vi "for testing.vi"() -> ()   [LabVIEW 2016]
uses:
  C:/Users/Anatec i3/Desktop/Labview Projects/IR OPO Controller/Branches/XPS version/uc480DotNet.dll
  uc480DotNet.dll
  <vilib>/Utility/miscctls.llb/LVBoundsTypeDef.ctl
  <vilib>/Utility/config.llb/Write Key (Double).vi
  <vilib>/Utility/config.llb/Write Key (I32).vi
  <vilib>/Utility/config.llb/Read Key (String).vi
  <vilib>/Utility/config.llb/Read Key (Double).vi
  <vilib>/Utility/config.llb/Read Key (I32).vi
  <vilib>/Utility/config.llb/NI_LVConfig.lvlib
  <vilib>/vision/NI_Vision_Development_Module.lvlib
  System.Windows.Forms
panel:
  out "[0]":i32
  out "x*y":dbl
  out "Image Pixels (U8)":u8[][](array[numeric])
  out "ROI width":dbl
  out "Lines":dbl
  out "height step size":dbl
  out "Xspot diam":dbl
  out "Y spot diam":dbl
  out "Process time":dbl=117.0
  in  "Width (µm)":i32=240
  in  "Y offset":i32=406 step=1
  in  "X offset":i32=693 step=1
  in  "Processing time unit":string(combo)="sec"
  in  "EXIT 2":bool
  in  "Camera":refnum<k24>(container)
  in  "Init Camera":bool
  in  "Start Live":bool
  in  "Stop Live":bool
  in  "Load Parameter":bool
  out "Error Out":errorcluster caption="error"
  out "Bits/Pixel":i32=32
  out "Width":i32=1280
  out "Height":i32=1024
  out "Serial Number":string="4102944807"
  in  "Camera ID":i32
  in  "Mode":i32(ring) items=["RGB 32"=0, "RGB 24"=1, "Y8 Monochrom"=6]
  in  "Zoom":dbl(ring)=1.5 items=["4X"=4.0, "2X"=2.0, "1.5X"=1.5, "1.25X"=1.25, "1X"=1.0]
  in  "Gain Boost":bool=TRUE
  in  "Snapshot":bool
  out "Output":picture
  out "Source":T1(plugin-control)
  in  "Exposure":dbl(slide)=99.80425000000001 min=0.06241666666666667 max=99.80425000000001 step=0.06241666666666667 scale=0.06241666666666667..99.80425000000001 scale format="%#.3g"
  in  "Framerate":dbl(slide)=10.002522802986672 min=0.47411700449083627 max=15.001275108384213 step=0.014032998230481021 scale=0.47411700449083627..15.001275108384213 scale format="%#.3g"
  in  "Pixelclock":i32(slide)=24 min=5 max=40 step=1 scale=5.0..40.0
  in  "Exit Camera":bool
  out "Camera Status":string="Load parameter"
  out "Log":string
  out "Y Step size in µm":i32=121
  out "Time array":dbl[][](array[numeric])
  out "ROI container\nheigth (µm)":i32=2267
  out "ROI container\nwidth (µm)":i32=2267
  out "Processi time (sec)":i32=117
  out "ROI Rectangle X position":i32=594
  out "Commands array":string[][](array[string])
  out "Laser on/off array":bool[][](array[boolean])
  out "ROI Area \n(mm2)":dbl=4.035870075999999
  out "Axis 1 Offset":dbl
  out "Axis 2 Offset":dbl
  out "ROI Rectangle Y Position":i32
  in  "Precision (%)":dbl=0.9 min=0.0 max=1.0 step=0.01 format="%#_13g"
  in  "Process Image":bool
  in  "EXIT 3":bool
  in  "Pixel size":dbl=12.19 step=0.01
  in  "Speed (µm/s)":i32=1000
  in  "Heigth (µm)":i32=240
  in  "Height  step \ndivider":i32=2
  in  "Wavelength":dbl=2940.0 min=2600.0 max=3200.0 step=1.0
  in  "Axis Initial Parameters":T2={"Velocity (units/seconds)"=1.0, "Acceleration (units/seconds²)"=20.0, "Minimum Jerk Time (seconds)"=0.005, "Maximum Jerk Time (seconds)"=0.009} {"Maximum Jerk Time (seconds)" format="%.6e"; "Minimum Jerk Time (seconds)" format="%.6e"; "Acceleration (units/seconds²)" format="%.6e"; "Velocity (units/seconds)" format="%.6e"}
  out "Axis 1":string
  out "Axis 2":string
  out "Default Wavelenght":i32
  out "XPS_Address":string
  out "Velocity":dbl
  out "Acceleration":dbl
  in  "Repetition \nRate":enum16{"1", "2", "5", "10", "20"}(ring)=enum."20"
  in  "Flash lamp - Q Switch delay (%)":i16(slide) min=0 max=100 scale=0.0..100.0 scale format="%#.1f"
  in  "Capture":bool
  in  "Log Capture":bool
  in  "Acceleration \n(mm/s²)":dbl=20.0
  in  "Transparency":u8 max=80 step=1
  in  "Home Axes":bool
  in  "Axes Manual Control":bool
  in  "Save configuration":bool
  in  "Stages status":bool
  in  "Open \nManual":bool
  in  "Alignment \ndiode":bool
  in  "Overlay MSI Image":bool
  in  "EXIT":bool
  in  "Tune":bool
  out "Laser Operation":bool
  in  "LASER":bool
  in  "LAMP":bool
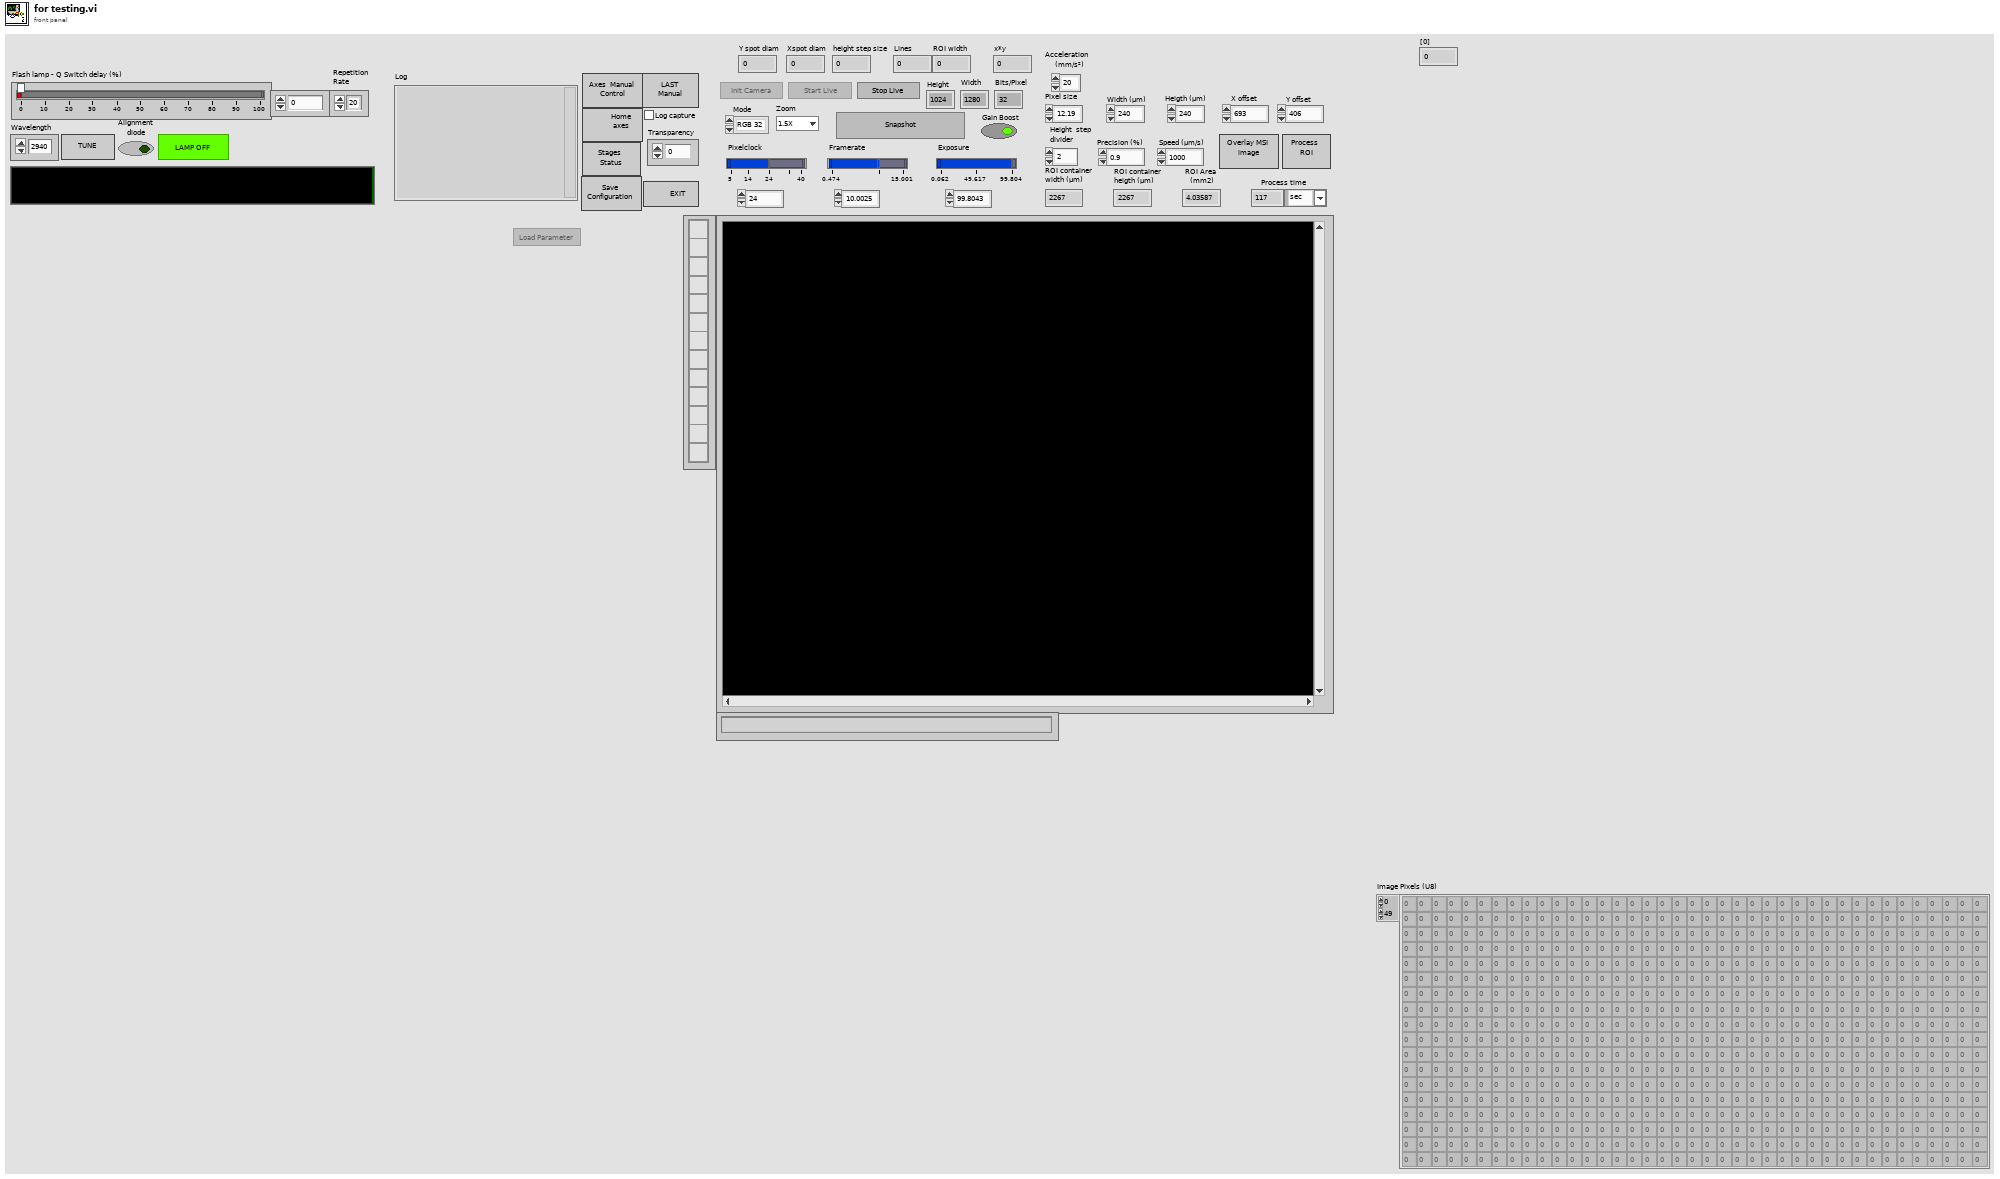
[diagram p1: front panel]
types:
  T1 = typedef "IMAQ Image.ctl" = refnum<image>
  T2 = cluster{"Velocity (units/seconds)":dbl, "Acceleration (units/seconds²)":dbl, "Minimum Jerk Time (seconds)":dbl, "Maximum Jerk Time (seconds)":dbl}
  T3 = typedef "Image Type" = u32
  T4 = cluster{"Global Rectangle":i32[], "Contours":cluster{"Contour Type":u32, "ROI Type":u32, "Points":i32[]}[]}
  T5 = typedef "NI_LVConfig.lvlib/Config Data RefNum.ctl" = refnum<k1>
  T6 = cluster{"connection TCP":refnum<k5>, "LogTo File":bool, "Log File refnum":refnum<file>, "no error if error log":bool}
  T7 = typedef "LVBoundsTypeDef.ctl" = cluster{"Width":u32, "Height":u32}
  T8 = enum8{"Enabled", "Disabled", "Disabled and Grayed Out"}
  T9 = enum16{"Initialize", "Lamp ON", "Lamp OFF", "Q-switch ON", "Q-switch OFF", "Adjust Energy", "Change Rep. Rate", "Send String"}
  T10 = enum16{"open", "replace", "create", "open or create", "replace or create", "replace or create with confirmation"}
  T11 = enum32{"Invalid", "Standard", "Closed", "Hidden", "Minimized", "Maximized"}
  T12 = enum32{"invalid app kind", "Development System", "Run Time System", "Student Edition", "Embedded LabVIEW", "Evaluation", "Custom"}
diagram:
  w16 = 1 items=["None", "FixedSingle", "Fixed3D"] ("BorderStyle")
  # "Camera control buttons"
  # "Button and controls"
  n1 = while "ROI Processing" {
    stop <- w52 stop-if-true
    n2 = event shown="[1] \"Process Image\": Value Change" {
      selector: _ -> [_ _]
      dyn-events: _ -> [_ _]
      timeout: _ -> [_ _]
      tunnel: ["EXIT 3" _] -> w52
      tunnel: [_ w58] -> w45
      event "EXIT": Value Change {
        n3 = event-data() -> ()  [unwired: 1 in, 6 out]
      }
      event "Process Image": Value Change {
        n4 = event-data() -> ()  [unwired: 1 in, 6 out]
        n5 = case shown="True" "Process Image" {
          tunnel: ["" "Processing done"] -> w58
          frame False {
          }
          frame True {
            w72 = 0.2  # Delay after laser on/off
            w84 = 2.0 ("y")
            w131 = T3 0 items=["Grayscale (U8)", "Grayscale (I16)", "Grayscale (SGL)", "Complex (CSG)", "RGB (U32)", "HSL (U32)", "RGB (U64)", "Grayscale (U16)"] ("Image Type")
            w134 = i16 3 ("precision (6)")
            w124 = 1000 ("y")
            n6 = local read "Source"() -> (w133:T1)
            n7 = property on="Source" class="ImageControl"() -> ("ROI"=w140:T4)  [unwired: 2 in, 2 out]
            n8 = call "IMAQ Cast Image"("Image Type"=w131, "Image Src"=w133) -> ("Image Dst Out"=w132:T1)  [unwired: 8 in, 1 out]
            n9 = Unbundle By Name(w140) -> ("Global Rectangle"=w139:i32[])
            n10 = call "IMAQ ROIToMask 2"("ROI Descriptor"=w140, "Image"=w132) -> ("Image Out"=w142:T1)  [unwired: 7 in, 2 out]
            n11 = local read "Heigth (µm)"() -> (w93:i32)
            n12 = local read "Width (µm)"() -> (w92:i32)
            n13 = local read "X offset"() -> (w127:i32)
            n14 = local read "Y offset"() -> (w129:i32)
            n15 = call "IMAQ ImageToArray"("Image"=w142) -> ("Image Pixels (U8)"=w114:u8[][])  [unwired: 3 in, 4 out]
            "Image Pixels (U8)" <- w114
            n16 = Index Array(array=w139, index=0) -> (element=w128:i32)
            "ROI Rectangle X position" <- w128
            n17 = Index Array(array=w139, index=1) -> (element=w130:i32)
            "ROI Rectangle Y Position" <- w130
            n18 = Divide "X spot radius in micron"(x=w92, y=w84) -> (x/y=w96:dbl)
            n19 = Divide "Y spot radius in micron"(x=w93, y=w84) -> (x/y=w95:dbl)
            n20 = Empty Array?(array=w114) -> (empty?=w115:bool)
            n21 = Subtract(x=w128, y=w127) -> (x-y=w136:i32)
            n22 = Subtract(x=w130, y=w129) -> (x-y=w135:i32)
            n23 = case shown="False" w115 {
              tunnel: [w172 u8[][] [[1]] ("Image Pixels (U8)")] -> w113
              tunnel: w114 -> [w172 _]
              frame False {
              }
              frame True {
                n24 = One Button Dialog(message="ATTENTION: you did not select\nany region of interest") -> ()  [unwired: 1 in, 1 out]
              }
            }
            n25 = local read "Pixel size"() -> (w104:dbl)
            n26 = Divide "X spot diameter in pixel"(x=w92, y=w104) -> (x/y=w63:dbl)
            "Xspot diam" <- w63
            n27 = Divide "Y spot diameter in pixel"(x=w93, y=w104) -> (x/y=w62:dbl)
            "Y spot diam" <- w62
            n28 = Multiply(x=w104, y=w104) -> (x*y=w118:dbl)
            n29 = Multiply(x=w136, y=w104) -> (x*y=w89:dbl)
            n30 = Multiply(x=w135, y=w104) -> (x*y=w97:dbl)
            n31 = Less Than 0?(x=w89) -> (x < 0?=w88:bool)
            n32 = Less Than 0?(x=w97) -> (x < 0?=w98:bool)
            n33 = Round To Nearest(number=w96) -> (nearest integer value=w90:dbl)
            n34 = Round To Nearest(number=w95) -> (nearest integer value=w91:dbl)
            n35 = local read "Height  step \ndivider"() -> (w145:i32)
            n36 = case shown="True" w88 {
              tunnel: w89 -> [w162 w165]
              tunnel: w90 -> [w161 w164]
              tunnel: [w160 w163] -> w87
              frame False {
                n37 = Subtract(x=w162, y=w161) -> (x-y=w160:dbl)
              }
              frame True {
                n38 = Add(x=w165, y=w164) -> (x+y=w163:dbl)
              }
            }
            n39 = case shown="False" w98 {
              tunnel: w97 -> [w168 w171]
              tunnel: w91 -> [w167 w170]
              tunnel: [w166 w169] -> w94
              frame False {
                n40 = Subtract(x=w168, y=w167) -> (x-y=w166:dbl)
              }
              frame True {
                n41 = Add(x=w171, y=w170) -> (x+y=w169:dbl)
              }
            }
            n42 = Divide "Y spot radius in pixels"(x=w62, y=w84) -> ()  [unwired: 1 out]
            n43 = Divide(x=w62, y=w145) -> (x/y=w100:dbl)
            n44 = Divide(x=w87, y=w124) -> (x/y=w126:dbl)
            n45 = Divide(x=w94, y=w124) -> (x/y=w125:dbl)
            n46 = Multiply "# pixels in an ablation spot"(x=w62, y=w63) -> (x*y=w65:dbl)
            "x*y" <- w65
            n47 = Round To Nearest(number=w100) -> (nearest integer value=w99:dbl)
            "height step size" <- w99
            n48 = Multiply(x=w104, y=w99) -> (x*y=→"Y Step size in µm":dbl)
            n49 = Array Size(array=w113) -> (size(s)=w143:i32[])
            n50 = To Double Precision Float(number=w113) -> (double precision float=w116:dbl[][])
            n51 = Number To Fractional String(number=w126, precision (6)=w134) -> (F-format string=w110:string)  [unwired: 2 in]
            n52 = Number To Fractional String(number=w125, precision (6)=w134) -> (F-format string=w111:string)  [unwired: 2 in]
            n53 = Add Array Elements(numeric array=w116) -> (sum=w120:dbl)
            n54 = Fract/Exp String To Number(string=w110) -> (number=→"Axis 1 Offset":dbl)  [unwired: 3 in, 1 out]
            n55 = Fract/Exp String To Number(string=w111) -> (number=→"Axis 2 Offset":dbl)  [unwired: 3 in, 1 out]
            n56 = Array To Cluster(array=w143) -> (cluster=w144:cluster{"[0]":i32, "[1]":i32})
            n57 = Unbundle(w144) -> ("[0]"=w61:i32, "[1]"=w66:i32)
            "[0]" <- w61
            n58 = Subtract(x=w66, y=w63) -> (x-y=w64:dbl)
            "ROI width" <- w64
            n59 = Divide(x=w120, y=u8 255) -> (x/y=w117:dbl)
            n60 = Divide "Total heigth lines"(x=w61, y=w99) -> (x/y=w112:dbl)
            n61 = Multiply(x=w117, y=w118) -> (x*y=w107:dbl)
            n62 = Multiply(x=w61, y=w104) -> (x*y=w102:dbl)
            n63 = Multiply(x=w66, y=w104) -> (x*y=w103:dbl)
            n64 = Round To Nearest(number=w102) -> (nearest integer value=→"ROI container\nheigth (µm)":dbl)
            n65 = Round To Nearest(number=w103) -> (nearest integer value=→"ROI container\nwidth (µm)":dbl)
            n66 = Divide(x=w107, y=1000000.0) -> (x/y=→"ROI Area \n(mm2)":dbl)
            n67 = Round To Nearest(number=w112) -> (nearest integer value=w86:dbl)
            "Lines" <- w86
            n68 = call "ROI parser.vi"("# pixels in an ablation spot"=w65, "ROI Height in pixel"=w86, "Heigth step size in pixel"=w99, "ROI (8 bit image)"=w113, "Ablation spot width"=w63, "ROI Width in pixel"=w64, "Sampling\nPrecision"="Precision (%)", "Ablation spot heigth"=w62) -> ("Parsed array"=w60:bool[][])  [unwired: 3 in]
            n69 = Index Array(array=w60, index (col)=0 ("disabled index (col)")) -> (element=w157:bool[])  [unwired: 1 in]
            n70 = Array Size(array=w157) -> (size(s)=w158:i32)
            n71 = call "Array processor.vi"("Source array"=w60, "Iterations"=w158) -> ("Lenght product array"=w156:i32[][], "T/F product array"=w79:bool[][])  [unwired: 8 in]
            n72 = for {
              tunnel: w156 -> [w179] mode=indexing
              tunnel: [w178] -> w141 mode=indexing
              # "This loop transform each lenght fragment into a µm size value"
              n73 = local read "Pixel size"() -> (w180:dbl)
              n74 = Multiply(x=w180, y=w179) -> (x*y=w178:dbl[])
            }
            n75 = Index Array(array=w79, index (col)=0 ("disabled index (col)")) -> (element=w148:bool[])  [unwired: 1 in]
            n76 = Array Size(array=w148) -> (size(s)=w147:i32)
            n77 = for {
              N: w147 -> [_]
              tunnel: w79 -> [w177] mode=indexing
              tunnel: [w175] -> w123 mode=indexing
              # "This loop add a F for each Y moviment"
              n78 = Build Array (concatenate)(w177, FALSE) -> (w175:bool[])
            }
            "Laser on/off array" <- w123
            n79 = local read "Y Step size in µm"() -> (w83:i32)
            n80 = local read "Speed (µm/s)"() -> (w80:i32)
            n81 = Index Array(array=w141, index (col)=0 ("disabled index (col)")) -> (element=w152:dbl[])  [unwired: 1 in]
            n82 = Index Array(array=w141, index (row)=0) -> (element=w154:dbl[])  [unwired: 1 in]
            n83 = Array Size(array=w152) -> (size(s)=w150:i32)
            n84 = Array Size(array=w154) -> (size(s)=w153:i32)
            n85 = local read "Axis 1"() -> (w82:string)
            n86 = local read "Axis 2"() -> (w81:string)
            n87 = call "Commands array generator.vi"("Axis 1"=w82, "Heigth"=w150, "Axis in"=w81, "Width"=w153, "Axes speed \n(µm/s)"=w80, "Y Step size in µm"=w83, "T/F product array"=w79, "Space defined array"=w141) -> ("Command Array"=→"Commands array":string[][], "Time Array"=w101:dbl[][])  [unwired: 2 in]
            "Time array" <- w101
            n88 = Array Size(array=w79) -> (size(s)=w78:i32[])
            n89 = Index Array(array=w78, index=0) -> (element=w75:i32)
            n90 = Index Array(array=w78, index=1) -> (element=w74:i32)
            n91 = Add Array Elements(numeric array=w101) -> (sum=w70:dbl)
            n92 = Multiply(x=w75, y=w74) -> (x*y=w73:i32)
            n93 = Multiply(x=w73, y=w72) -> (x*y=w71:dbl)
            n94 = Add(x=w71, y=w70) -> (x+y=w69:dbl)
            "Processi time (sec)" <- w69
            n95 = local write "Process time"(w69) -> ()
          }
        }
      }
    }
    n96 = Get Date/Time In Seconds() -> (seconds since 1Jan1904=w48:timestamp)
    n97 = Format Date/Time String(time format string (%c)="%m/%d/%y - %I:%M %p  ", seconds (now)=w48) -> (date/time string=w47:string)  [unwired: 1 in]
    n98 = Empty String/Path?(string/path=w45) -> (empty?=w46:bool)
    n99 = Concatenate Strings(w47, w45, "\r") -> (w51:string)
    n100 = case shown="False" w46 {
      tunnel: w51 -> [w55 _]
      frame False {
        n101 = invoke on="Log" class="Str" method="Append String"("string"=w55) -> (error out=w53:errorcluster)  [unwired: 3 in, 3 out]
        n102 = property on="Log" class="Str"(error in=w53, "Text.Scroll Position"=u32 500000) -> ()  [unwired: 1 in, 2 out]
      }
      frame True {
      }
    }
  }
  n103 = flat-sequence "Initialization sequence" {
    tunnel: [w197] -> w44
    tunnel: w44 -> [w259]
    tunnel: [w242] -> w42
    tunnel: [w241] -> w41
    tunnel: [w240] -> w43
    tunnel: [w239] -> w40
    tunnel: [w238] -> w39
    tunnel: w43 -> [w270]
    tunnel: w42 -> [w269]
    tunnel: w41 -> [w268]
    tunnel: [w267] -> w38
    tunnel: w40 -> [w266]
    tunnel: w39 -> [w265]
    tunnel: [w262] -> w37
    tunnel: [w261] -> w36
    tunnel: w38 -> [w290]
    tunnel: [w290] -> w35
    tunnel: w37 -> [w289]
    tunnel: [w288] -> w34
    tunnel: w36 -> [w288]
    tunnel: w35 -> [w300]
    tunnel: [w300] -> w33
    tunnel: w34 -> [w299]
    tunnel: [w309] -> w32
    tunnel: w33 -> [w309]
    tunnel: [w310] -> w31
    tunnel: w32 -> [w310]
    tunnel: [w319] -> w30
    tunnel: w31 -> [w319]
    tunnel: [w320] -> w29
    tunnel: w30 -> [w320]
    tunnel: w29 -> [w322]
    tunnel: [w322] -> w28
    tunnel: w28 -> [w324]
    tunnel: [w324] -> w27
    tunnel: w27 -> [w326]
    tunnel: [w326] -> w26
    tunnel: w26 -> [w327]
    frame #0 {
      w181 = FALSE ("Visible")
      n104 = control-ref of="This VI"() -> (w182:refnum<vi>)
      n105 = invoke class="VI" method="Default Vals.Reinit All"(reference=w182) -> ()  [unwired: 2 in, 3 out]
      n106 = property on="Axes Manual Control" class="Bool (strict)"("Visible"=w181) -> ()  [unwired: 2 in, 2 out]
      n107 = property on="Home Axes" class="Bool"("Visible"=w181) -> ()  [unwired: 2 in, 2 out]
    }
    frame #1 {
      w215 = "ROI Processing" ("section")
      w223 = "XPS" ("section")
      n108 = control-ref of="This VI"() -> (w237:refnum<vi>)
      n109 = property class="VI"(reference=w237) -> ("Path"=w235:path)  [unwired: 1 in, 2 out]
      n110 = Strip Path(path=w235) -> (stripped path=w234:path)  [unwired: 1 out]
      n111 = Build Path(base path=w234, name or relative path="General_Configuration.ini") -> (appended path=w225:path)
      n112 = call <vilib>:"Open Config Data.vi"("create file if necessary (T)"=FALSE, "configuration file path"=w225) -> ("error out"=w224:errorcluster, "refnum"=w196:T5)  [unwired: 7 in, 1 out]
      n113 = call-poly <vilib>:"Read Key.vi"("section"="Communication", "default value"="192.168.254.254", "key"="XPSPort", "refnum"=w196) -> ("error out"=w190:errorcluster, "value"=→"XPS_Address":string)  [unwired: 4 in, 2 out]
      n114 = call-poly <vilib>:"Read Key.vi"("section"=w223, "error in (no error)"=w224, "default value"=1.0, "key"="InitialVelocity", "refnum"=w196) -> ("error out"=w189:errorcluster, "value"=→"Velocity":dbl)  [unwired: 3 in, 2 out]
      n115 = call-poly <vilib>:"Read Key.vi"("section"=w223, "default value"=20.0, "key"="Acceleration", "refnum"=w196) -> ("error out"=w188:errorcluster, "value"=→"Acceleration":dbl)  [unwired: 4 in, 2 out]
      n116 = call-poly <vilib>:"Read Key.vi"("section"="Laser" ("key"), "default value"=0, "key"="Wavelenght", "refnum"=w196) -> ("error out"=w187:errorcluster, "value"=→"Default Wavelenght":i32)  [unwired: 4 in, 2 out]
      n117 = Merge Errors(w190, w189, w188, w187) -> (w191:errorcluster)
      n118 = call-poly <vilib>:"Read Key.vi"("section"=w215, "key"="Pixel Size", "refnum"=w196) -> ("error out"=w206:errorcluster, "value"=w195:dbl)  [unwired: 5 in, 2 out]
      n119 = call-poly <vilib>:"Read Key.vi"("section"=w215, "key"="Heigth step divider", "refnum"=w196) -> ("error out"=w205:errorcluster, "value"=w194:i32)  [unwired: 5 in, 2 out]
      n120 = call-poly <vilib>:"Read Key.vi"("section"=w215, "key"="Precision (%)", "refnum"=w196) -> ("error out"=w204:errorcluster, "value"=w192:dbl)  [unwired: 5 in, 2 out]
      n121 = call-poly <vilib>:"Read Key.vi"("section"=w215, "key"="Sampling speed", "refnum"=w196) -> ("error out"=w203:errorcluster, "value"=w193:i32)  [unwired: 5 in, 2 out]
      n122 = call-poly <vilib>:"Read Key.vi"("section"=w215, "key"="Width", "refnum"=w196) -> ("error out"=w202:errorcluster, "value"=w186:i32)  [unwired: 5 in, 2 out]
      n123 = call-poly <vilib>:"Read Key.vi"("section"=w215, "key"="Height", "refnum"=w196) -> ("error out"=w201:errorcluster, "value"=w185:i32)  [unwired: 5 in, 2 out]
      n124 = call-poly <vilib>:"Read Key.vi"("section"=w215, "key"="X offset", "refnum"=w196) -> ("error out"=w200:errorcluster, "value"=w184:i32)  [unwired: 5 in, 2 out]
      n125 = call-poly <vilib>:"Read Key.vi"("section"=w215, "key"="Y offset", "refnum"=w196) -> ("error out"=w199:errorcluster, "value"=w183:i32)  [unwired: 5 in, 2 out]
      n126 = Merge Errors(w206, w205, w204, w203, w202, w201, w200, w199, w191) -> (w198:errorcluster)
      n127 = local write "Height  step \ndivider"(w194) -> ()
      n128 = call <vilib>:"Close Config Data.vi"("error in (no error)"=w198, "refnum"=w196) -> ("error out"=w197:errorcluster)  [unwired: 8 in, 1 out]
      n129 = local write "Speed (µm/s)"(w193) -> ()
      n130 = local write "Precision (%)"(w192) -> ()
      n131 = local write "Pixel size"(w195) -> ()
      n132 = local write "Heigth (µm)"(w185) -> ()
      n133 = local write "Width (µm)"(w186) -> ()
      n134 = local write "Y offset"(w183) -> ()
      n135 = local write "X offset"(w184) -> ()
    }
    frame #2 {
      w243 = "\r"
      n136 = local read "XPS_Address"() -> (w260:string)
      n137 = call <userlib>:"Open TCP-IP.vi"("error in (no error)"=w259, "IP address"=w260) -> ("error out"=w257:errorcluster, "Connection ID"=w258:T6)  [unwired: 4 in, 4 out]
      n138 = call <userlib>:"Objects List Get.vi"("error in (no error)"=w257, "connection ID in"=w258) -> ("error out"=w238:errorcluster, "XPS error out"=w239:errorcluster, "connection ID out"=w240:T6, "Groups"=w256:string[])  [unwired: 4 in, 2 out]
      n139 = Get Date/Time In Seconds() -> (seconds since 1Jan1904=w252:timestamp)
      n140 = Format Date/Time String(time format string (%c)="%m/%d/%y -%I:%M %p  ", seconds (now)=w252) -> (date/time string=w245:string)  [unwired: 1 in]
      n141 = Index Array(array=w256) -> (element=w241:string)  [unwired: 1 in]
      "Axis 1" <- w241
      n142 = Index Array(array=w256, index=1) -> (element=w242:string)
      "Axis 2" <- w242
      n143 = Concatenate Strings(w245, "Axis 1: " ("Initialiazation"), w241, w243) -> (w254:string)
      n144 = Concatenate Strings(w245, "Axis 2: " ("Initialiazation"), w242, w243) -> (w246:string)
      n145 = invoke on="Log" class="Str" method="Append String"("string"=w254) -> (error out=w250:errorcluster)  [unwired: 3 in, 3 out]
      n146 = invoke on="Log" class="Str" method="Append String"("string"=w246) -> (error out=w247:errorcluster)  [unwired: 3 in, 3 out]
      n147 = property on="Log" class="Str"(error in=w250, "Text.Scroll Position"=u32 500000) -> ()  [unwired: 1 in, 2 out]
      n148 = property on="Log" class="Str"(error in=w247, "Text.Scroll Position"=u32 500000) -> ()  [unwired: 1 in, 2 out]
    }
    frame #3 {
      w284 = "Ready"
      n149 = call "Get Stages Status.vi"("error in (no error)"=w265, "XPS error in (no error)"=w266, "Group Name (250 c max)"=w268, "connection ID in"=w270) -> ("error out"=w275:errorcluster, "XPS error out"=w276:errorcluster, "Group Status String"=w272:string, "connection ID out"=w277:T6)  [unwired: 3 in, 1 out]
      n150 = call "Get Stages Status.vi"("error in (no error)"=w275, "XPS error in (no error)"=w276, "Group Name (250 c max)"=w269, "connection ID in"=w277) -> ("error out"=w273:errorcluster, "XPS error out"=w263:errorcluster, "Group Status String"=w271:string, "connection ID out"=w274:T6)  [unwired: 3 in, 1 out]
      n151 = String Subset(string=w272, offset (0)=0, length (rest)=5 ("length (rest)")) -> (substring=w282:string)
      n152 = Bundle(cluster="Axis Initial Parameters", "Velocity (units/seconds)"=5.0) -> (w286:T2)  [unwired: 3 in]
      n153 = call <userlib>:"Close TCP-IP.vi"("error in (no error)"=w273, "connection ID in"=w274) -> ("Error out"=w264:errorcluster)  [unwired: 9 in]
      n154 = local write "Axis Initial Parameters"(w286) -> ()
      n155 = String Subset(string=w271, offset (0)=0, length (rest)=5 ("length (rest)")) -> (substring=w283:string)
      n156 = call <vilib>:"Simple Error Handler.vi"("error in (no error)"=w264) -> ()  [unwired: 4 in, 5 out]
      n157 = call <vilib>:"Simple Error Handler.vi"("error in (no error)"=w263) -> ()  [unwired: 4 in, 5 out]
      n158 = Equal?(x=w282, y=w284) -> (x = y?=w262:bool)
      n159 = Equal?(x=w284, y=w283) -> (x = y?=w261:bool)
      n160 = And(x=w262, y=w261) -> (x .and. y?=w267:bool)
    }
    frame #4 {
      n161 = case shown="True" w289 {
        frame False {
        }
        frame True {
          (unwired) u32 500000 ("Text.Scroll Position")
          n162 = Get Date/Time In Seconds() -> (seconds since 1Jan1904=w295:timestamp)
          n163 = Format Date/Time String(time format string (%c)="%m/%d/%y -%I:%M %p  ", seconds (now)=w295) -> (date/time string=w294:string)  [unwired: 1 in]
          n164 = Concatenate Strings(w294, "Axis 1 ready" ("Initialiazation"), "\r") -> (w292:string)
          n165 = invoke on="Log" class="Str" method="Append String"("string"=w292) -> (error out=w293:errorcluster)  [unwired: 3 in, 3 out]
          n166 = property on="Log" class="Str"(error in=w293, "Text.Scroll Position"=u32 500000) -> ()  [unwired: 1 in, 2 out]
        }
      }
    }
    frame #5 {
      n167 = case shown="True" w299 {
        frame False {
        }
        frame True {
          (unwired) u32 500000 ("Text.Scroll Position")
          n168 = Get Date/Time In Seconds() -> (seconds since 1Jan1904=w305:timestamp)
          n169 = Format Date/Time String(time format string (%c)="%m/%d/%y -%I:%M %p  ", seconds (now)=w305) -> (date/time string=w304:string)  [unwired: 1 in]
          n170 = Concatenate Strings(w304, "Axis 2 enabled" ("Initialiazation"), "\r") -> (w302:string)
          n171 = invoke on="Log" class="Str" method="Append String"("string"=w302) -> (error out=w303:errorcluster)  [unwired: 3 in, 3 out]
          n172 = property on="Log" class="Str"(error in=w303, "Text.Scroll Position"=u32 500000) -> ()  [unwired: 1 in, 2 out]
        }
      }
    }
    frame #6 {
    }
    frame #7 {
      w316 = FALSE ("Visible")
      # "Set defaults"
      n173 = local write "Flash lamp - Q Switch delay (%)"(i16 0 ("Energy")) -> ()
      n174 = local write "Alignment \ndiode"(TRUE ("Alignment diode")) -> ()
      n175 = local write "Repetition \nRate"(enum16{"1", "2", "5", "10", "20"}."20" ("Rep. Rate Divider")) -> ()
      n176 = call "IR_Alignment_Diode.vi"("AD Action"=enum16{"AD Off", "AD On"}."AD On") -> ()  [unwired: 14 in, 1 out]
      n177 = property on="LAMP" class="Bool (strict)"("BoolText.Text"="LAMP OFF" ("Boolean Text.Text")) -> ()  [unwired: 2 in, 2 out]
      n178 = property on="Laser Operation" class="Bool (strict)"("Blinking"=w316) -> ()  [unwired: 2 in, 2 out]
      n179 = property on="Capture" class="Bool"("Visible"=w316) -> ()  [unwired: 2 in, 2 out]
      n180 = property on="LASER" class="Bool (strict)"("BoolText.Text"="LASER OFF" ("Boolean Text.Text"), "Visible"=FALSE) -> ()  [unwired: 2 in, 2 out]
    }
    frame #8 {
    }
    frame #9 {
    }
    frame #10 {
      n181 = local write "Camera Status"("Init camera" ("Camera Status")) -> ()
    }
    frame #11 {
      n182 = Wait (ms)(milliseconds to wait=u32 1000) -> ()  [unwired: 1 out]
    }
    frame #12 {
      n183 = local write "Camera Status"("Start live") -> ()
    }
    frame #13 {
      n184 = case shown="True" w327 {
        frame False {
          n185 = One Button Dialog(message="Axes not ready") -> ()  [unwired: 1 in, 1 out]
        }
        frame True {
          n186 = Get Date/Time In Seconds() -> (seconds since 1Jan1904=w334:timestamp)
          n187 = property on="Home Axes" class="Bool"("Visible"=TRUE) -> ()  [unwired: 2 in, 2 out]
          n188 = property on="Axes Manual Control" class="Bool (strict)"("Visible"=TRUE) -> ()  [unwired: 2 in, 2 out]
          n189 = Format Date/Time String(time format string (%c)="%m/%d/%y -%I:%M %p  ", seconds (now)=w334) -> (date/time string=w335:string)  [unwired: 1 in]
          n190 = Concatenate Strings(w335, "System ready" ("Initialiazation"), "\r") -> (w337:string)
          n191 = invoke on="Log" class="Str" method="Append String"("string"=w337) -> (error out=w336:errorcluster)  [unwired: 3 in, 3 out]
          n192 = property on="Log" class="Str"(error in=w336, "Text.Scroll Position"=u32 500000) -> ()  [unwired: 1 in, 2 out]
        }
      }
    }
  }
  n193 = property class="PictureBox"(reference="Camera", "BorderStyle"=w16, "Width"=853, "Height"=682) -> (reference out=w4:refnum<k24>, error out=w5:errorcluster)  [unwired: 1 in]
  n194 = property class="PictureBox"(reference=w4, error in=w5) -> (reference out=w3:refnum<k24>, error out=w2:errorcluster, "Handle"=w1:refnum<k24>)
  n195 = while "Camera Control" {
    shift-right: [w346] -> _
    shift-left: w2 -> [w352]
    shift-right: [w349] -> _
    shift-left: _ -> [w342]
    shift-right: [w344] -> _
    shift-left: w3 -> [w345]
    tunnel: w1 -> [w343]
    stop <- w350 stop-if-true
    # ".NetReference"
    # ".Net Reference"
    n196 = event shown="[1] Timeout" {
      selector: _ -> [_ _]
      dyn-events: _ -> [_ _]
      timeout: 0 -> [_ _]
      event "Load Parameter", "Start Live": Mouse Down {
        n197 = event-data() -> ()  [unwired: 1 in, 2 out]
      }
      event Timeout {
        n198 = event-data() -> ()  [unwired: 1 in, 2 out]
      }
    }
    n199 = event shown="[1] Timeout" {
      selector: _ -> [_ _]
      dyn-events: _ -> [_ _]
      timeout: 0 -> [_ _]
      tunnel: [w366 w377] -> w353
      tunnel: w352 -> [w376 w377]
      tunnel: w342 -> [w375 _]
      event "Pixelclock": Value Change; "Pixelclock": Mouse Move; "Pixelclock": Key Down; "Pixelclock": Mouse Up {
        n200 = event-data() -> ("CtlRef"=w368:refnum<vi>)  [unwired: 1 in, 3 out]
        n201 = call "uc480_SubVI_Example_GetFramerate.vi"(".NET (Reference)"=w375, "Error In"=w376) -> ("Framerate"=w374:dbl, "Inc"=w373:dbl, "Min"=w371:dbl, "Max"=w372:dbl, "error out"=w370:errorcluster)  [unwired: 9 in]
        n202 = property on="Framerate" class="Slide (strict)"(error in=w370, "Value"=w374, "Increment"=w373, "Minimum"=w371, "Maximum"=w372) -> (error out=w369:errorcluster)  [unwired: 1 in, 1 out]
        n203 = property on="Framerate" class="Slide (strict)"(error in=w369, "Scale.Increment"=w373, "Scale.Minimum"=w371, "Scale.Maximum"=w372) -> (error out=w367:errorcluster)  [unwired: 1 in, 1 out]
        n204 = Close Reference(reference=w368, error in (no error)=w367) -> (error out=w366:errorcluster)
      }
      event Timeout {
        n205 = event-data() -> ()  [unwired: 1 in, 2 out]
      }
    }
    n206 = case shown="False" "Load Parameter" {
      tunnel: ["" "Load parameter"] -> w359
      frame False {
      }
      frame True {
      }
    }
    n207 = case shown="False" "Init Camera" {
      tunnel: ["" "Init camera"] -> w363
      frame False {
      }
      frame True {
      }
    }
    n208 = case shown="False" "Exit Camera" {
      tunnel: ["" "Exit camera"] -> w357
      frame False {
      }
      frame True {
      }
    }
    n209 = event shown="[1] Timeout" {
      selector: _ -> [_ _]
      dyn-events: _ -> [_ _]
      timeout: 0 -> [_ _]
      tunnel: w353 -> [w388 w389]
      tunnel: [w378 w389] -> w355
      tunnel: w342 -> [w387 _]
      event "Pixelclock", "Framerate": Value Change; "Pixelclock", "Framerate": Mouse Move; "Pixelclock", "Framerate": Key Down; "Pixelclock", "Framerate": Mouse Up {
        n210 = event-data() -> ("CtlRef"=w380:refnum<vi>)  [unwired: 1 in, 3 out]
        n211 = call "uc480_SubVI_Example_GetExposure.vi"(".NET (Reference)"=w387, "Error In"=w388) -> ("Exposure"=w384:dbl, "Inc"=w383:dbl, "Min"=w382:dbl, "Max"=w381:dbl, "Error out"=w385:errorcluster)  [unwired: 9 in]
        n212 = property on="Exposure" class="Slide (strict)"(error in=w385, "Value"=w384, "Increment"=w383, "Minimum"=w382, "Maximum"=w381) -> (error out=w386:errorcluster)  [unwired: 1 in, 1 out]
        n213 = property on="Exposure" class="Slide (strict)"(error in=w386, "Scale.Increment"=w383, "Scale.Minimum"=w382, "Scale.Maximum"=w381) -> (error out=w379:errorcluster)  [unwired: 1 in, 1 out]
        n214 = Close Reference(reference=w380, error in (no error)=w379) -> (error out=w378:errorcluster)
      }
      event Timeout {
        n215 = event-data() -> ()  [unwired: 1 in, 2 out]
      }
    }
    n216 = case shown="False" "Start Live" {
      tunnel: ["" "Start live"] -> w362
      frame False {
      }
      frame True {
      }
    }
    n217 = case shown="False" "Stop Live" {
      tunnel: ["" "Stop live"] -> w358
      frame False {
      }
      frame True {
      }
    }
    n218 = local read "Camera Status"() -> (w339:string)
    n219 = Concatenate Strings(w363, w362, w359, w358, w357) -> (→"Camera Status":string)
    n220 = case shown="Default" w339 {
      tunnel: w342 -> [w432 w472 w530 w572 w752 w811]
      tunnel: w355 -> [w435 w473 w531 w582 w751 w812]
      tunnel: [w406 w471 w539 w581 w710 w810] -> w349
      tunnel: [w407 w470 w540 w580 w747 w808] -> w348
      tunnel: [FALSE FALSE TRUE FALSE FALSE FALSE] -> w350
      tunnel: w345 -> [w405 w464 w512 w564 w705 w801]
      tunnel: [w405 w464 w511 w563 w705 w801] -> w344
      tunnel: w343 -> [_ _ _ w560 _ _]
      frame "Load parameter" {
        # "SubVI Example for \nMemory allocation"
        # "Is acquisition running?"
        # "Load Parameter"
        n221 = property class="Camera"(reference=w432, error in=w435) -> (error out=w440:errorcluster, "Acquisition"=w439:refnum<k24>)  [unwired: 1 out]
        n222 = invoke class="Acquisition" method="HasStarted"(reference=w439, error in=w440) -> (reference out=w436:refnum<k24>, error out=w438:errorcluster, "bValue"=w434:bool)  [unwired: 2 in, 1 out]
        n223 = control-ref of="Start Live"() -> (w430:refnum<vi>)
        n224 = invoke class="Acquisition" method="ToString"(reference=w436, error in=w438) -> (reference out=w402:refnum<k24>, error out=w401:errorcluster, "ToString"=w437:string)  [unwired: 1 in]
        n225 = property class="Bool"(reference=w430, "Disabled"=u8 0 ("Deaktiviert")) -> (reference out=w404:refnum<vi>, error out=w403:errorcluster)  [unwired: 1 in]
        n226 = Close Reference(reference=w402, error in (no error)=w401) -> (error out=w400:errorcluster)
        n227 = Close Reference(reference=w404, error in (no error)=w403) -> ()  [unwired: 1 out]
        n228 = call "uc480_Error_Handling.vi"("Error String"=w437, "Error In"=w400) -> ("Error Out"=w433:errorcluster)  [unwired: 9 in]
        n229 = case shown="False" w434 {
          tunnel: w433 -> [w448 w455]
          tunnel: w432 -> [w446 w456]
          tunnel: [w447 w455] -> w431
          tunnel: [w446 w456] -> w406
          frame False {
            n230 = property class="Camera"(reference=w446, error in=w448) -> (error out=w450:errorcluster, "Parameter"=w449:refnum<k24>)  [unwired: 1 out]
            n231 = invoke class="Parameter" method="Load"(reference=w449, error in=w450, "strFilename"="") -> (reference out=w452:refnum<k24>, error out=w453:errorcluster, "Load"=w445:i32)  [unwired: 1 in, 1 out]
            n232 = invoke class="Parameter" method="ToString"(reference=w452, error in=w453) -> (reference out=w442:refnum<k24>, error out=w444:errorcluster, "ToString"=w454:string)  [unwired: 1 in]
            n233 = Close Reference(reference=w442, error in (no error)=w444) -> (error out=w443:errorcluster)